vi "HFRR ADV v038 new software.vi"() -> ()   [LabVIEW 2025] (continued)
        n1697 = call <vilib>:"Clear Errors.vi"("error in (no error)"=w2110) -> ()  [unwired: 5 in, 2 out]
        n1698 = local write "Port 2a"(FALSE ("Port 2a")) -> ()
        n1699 = local read "Com Port 2"() -> (w2103:refnum<visa-resource-name>)
        "visa due" <- w2103
        n1700 = call-poly "VISA Configure Serial Port"("VISA resource name"=w2103, "timeout (10sec)"=w2114, "baud rate (9600)"=u32 250000 ("baud rate  2"), "data bits (8)"=u16 8 ("data bits  2"), "parity (0:none)"=w2113, "stop bits (10: 1 bit)"=w2115, "flow control (0:none)"=w2117) -> ("VISA resource name out"=w2118:refnum<visa-resource-name>, "error out"=w2119:errorcluster)  [unwired: 7 in]
        n1701 = flat-sequence {
          tunnel: w2118 -> [w2121]
          tunnel: w2119 -> [w2120]
          tunnel: [w2121] -> w2111
          tunnel: [w2120] -> w2104
          frame #0 {
            n1702 = Wait (ms)(milliseconds to wait=u32 50) -> ()  [unwired: 1 out]
          }
        }
        "Residual Due" <- ""
      }
    }
    "error out 9" <- w2045
    n1703 = local read "Quit"() -> (w2047:bool)
    "Error Due" <- w2052
  }
  n1704 = local write "FRICVALZ"(0.0 ("FRICVALZ")) -> ()
  n1705 = property on="RUN" class="Bool (strict)"("Visible"=TRUE) -> ()  [unwired: 2 in, 2 out]
  n1706 = while {
    tunnel: [w2136] -> _
    tunnel: [w2123] -> w54
    i -> [w2136]
    stop <- w2123 stop-if-true
    n1707 = local read "conststatus"() -> (w2127:dbl)
    n1708 = local read "Main Tab"() -> (w2125:T2)
    n1709 = local read "EDIT"() -> (w2142:bool)
    n1710 = local read "Rate"() -> (w2141:dbl)
    n1711 = case shown="True" w2142 {
      tunnel: [FALSE TRUE] -> _
      frame False {
      }
      frame True {
      }
    }
    n1712 = Equal?(x=w2125, y=T28."About" ("Main Tab")) -> (x = y?=w2134:bool)
    n1713 = Equal?(x=w2127, y=0.0) -> (x = y?=w2128:bool)
    n1714 = Divide(x=1.0, y=w2141) -> (x/y=w2137:dbl)
    "Time 2" <- w2137
    n1715 = case shown="True" w2128 {
      frame False {
      }
      frame True {
        # "C:\\WinDucom\\calibrate WO 2391.dcf"
        n1716 = local write "Lan flag"(22) -> ()
        n1717 = local write "conststatus"(10.0 ("rpm value : 2")) -> ()
        n1718 = String To Path(string="C:\\LAB-IQ\\calibrate WO 2465.dcf") -> (path=w2148:path)
        n1719 = Open/Create/Replace File "Open File"(file path (use dialog)=w2148) -> (refnum out=w2146:refnum<file>)  [unwired: 5 in, 2 out]
        n1720 = for {
          N: 23 -> [_]
          tunnel: w2146 -> [w2157]
          i -> [w2151]
          (unwired) TRUE ("line mode (F)")
          n1721 = Read from Text File "Read File"(file (use dialog)=w2157) -> (text=w2156:string)  [unwired: 3 in, 3 out]
          n1722 = Match Pattern(string=w2156, regular expression="]") -> (after substring=w2154:string)  [unwired: 1 in, 3 out]
          n1723 = String Subset(string=w2156, offset (0)=5, length (rest)=10 ("length (rest)")) -> (substring=w2149:string)
          n1724 = Fract/Exp String To Number(string=w2149) -> (number=w2150:dbl)  [unwired: 3 in, 1 out]
          n1725 = Match Pattern(string=w2154, regular expression="-") -> (before substring=w2152:string)  [unwired: 1 in, 3 out]
          n1726 = case shown="10" w2151 {
            tunnel: w2150 -> [_ _ _ _ _ _ _ _ _ _ w2164 _ _ _ _ _ _ _ _ _ _ _ _ _]
            tunnel: w2152 -> [_ _ _ _ w2160 w2161 w2162 _ _ _ _ _ _ _ _ _ _ _ _ _ w2165 w2166 w2167 _]
            frame 0 {
            }
            frame 1 {
            }
            frame 2 {
            }
            frame 3 {
            }
            frame 4 {
              n1727 = local write "Com Port 1"(w2160) -> ()
            }
            frame 5 {
              n1728 = local write "Com Port 2"(w2161) -> ()
              n1729 = local write "visa due"(w2161) -> ()
            }
            frame 6 {
              n1730 = String To Path(string=w2162) -> (path=w2163:path)
              n1731 = local write "File Path"(w2163) -> ()
              "String" <- w2162
            }
            frame 7 {
            }
            frame 8 {
            }
            frame 9 {
            }
            frame 10 {
              n1732 = local write "Language Selection"(w2164) -> ()
            }
            frame 11 {
            }
            frame 12 {
            }
            frame 13 {
            }
            frame 14 {
            }
            frame 15 {
            }
            frame 16 {
            }
            frame 17 {
            }
            frame 18 {
            }
            frame 21 {
            }
            frame 22 {
              n1733 = local write "Com Port 3"(w2165) -> ()
            }
            frame 20 {
              n1734 = local write "Camera Port :"(w2166) -> ()
            }
            frame 19 {
              n1735 = local write "C3 :"(w2167) -> ()
            }
            frame 23, Default {
            }
          }
        }
      }
    }
    n1736 = Select(t=u32 2500 ("milliseconds to wait"), s=w2134, f=u32 500 ("milliseconds to wait")) -> (s? t:f=w2132:u32)
    n1737 = Multiply(x=w2137, y=w2132) -> (x*y=w2139:dbl)
    n1738 = call "Elapsed Time2"("Time Target (s)"=w2139, "Auto Reset"=TRUE) -> ("Time has Elapsed"=w2129:bool)  [unwired: 10 in, 7 out]
    n1739 = case shown="True" w2129 {
      frame False {
      }
      frame True {
        n1740 = stacked-sequence {
          frame #0 {
            # "DATA PROCESSING"
            # "115 mV/N"
            n1741 = local read "Sample Temperature"() -> (w2170:dbl)
            n1742 = local read "RH Numeric:"() -> (→"Humidity ( %RH )" →"Hum":dbl)
            n1743 = local read "FRICVALZ"() -> (w2187:dbl)
            n1744 = local read "Friction"() -> (w2173:dbl)
            n1745 = call <vilib>:"Mean PtByPt.vi"("x"=w2170, "sample length"=100) -> ("mean"=w2169:dbl)  [unwired: 2 in, 1 out]
            "TEMP 2" <- w2169
            "TEMP 3" <- w2169
            n1746 = Subtract(x=w2173, y=w2187) -> (x-y=w2182:dbl)
            "FF 2" <- w2182
            "FF 4" <- w2182
            n1747 = local read "Ambient Temperature"() -> (→"AIR TEMP":dbl)
            n1748 = local read "TEMP"() -> (w2186:dbl)
            n1749 = local write "FF 3"(w2182) -> ()
            n1750 = Compound Arithmetic op=OR("FRICVALZ 4", "FRICVALZ 3", "FRICVALZ 2") -> (w2178:bool)
            n1751 = case shown="True" w2178 {
              tunnel: w2173 -> [_ w2193]
              frame False {
              }
              frame True {
                w2192 = FALSE ("FRICVALZ")
                n1752 = local write "FRICVALZ 3"(w2192) -> ()
                n1753 = local write "FRICVALZ 2"(w2192) -> ()
                n1754 = local write "FRICVALZ 4"(w2192) -> ()
                "FRICVALZ" <- w2193
              }
            }
            n1755 = Not A Number/Path/Refnum?(number/path/refnum=w2186) -> (NaN/Path/Refnum?=w2185:bool)
            n1756 = Not A Number/Path/Refnum?(number/path/refnum=w2182) -> (NaN/Path/Refnum?=w2184:bool)
            n1757 = Divide(x=w2182, y=1.96) -> (x/y=w2179:dbl)
            n1758 = Compound Arithmetic op=OR(w2185, w2184) -> (w2183:bool)
            n1759 = Not A Number/Path/Refnum?(number/path/refnum=w2179) -> (NaN/Path/Refnum?=w2180:bool)
            n1760 = case shown="True" w2183 {
              frame False {
              }
              frame True {
                n1761 = local write "TEMP"(0.0 ("TEMP")) -> ()
                n1762 = local write "FF 2"(0.0 ("FF 2")) -> ()
                n1763 = local write "reinit"(TRUE ("reinit")) -> ()
              }
            }
            n1764 = local write "TEMP"(w2169) -> ()
            n1765 = Select(t=0.0, s=w2180, f=w2179) -> (s? t:f=w2172:dbl)
            "COF 2" <- w2172
            n1766 = local write "COF 3"(w2172) -> ()
          }
        }
      }
    }
    n1767 = Wait (ms)(milliseconds to wait=u32 50) -> ()  [unwired: 1 out]
    n1768 = local read "Quit"() -> (w2123:bool)
    "Rate" <- 2500.0 ("No of Samples")
  }
  n1769 = while {
    tunnel: [w2213] -> _
    tunnel: [w2196] -> w56
    tunnel: w1 -> [_]
    i -> [w2213]
    stop <- w2196 stop-if-true
    # "C:\\LAB-IQ-NXT\\Scar View.exe"
    n1770 = local read "OK Button 16"() -> (w2203:bool)
    n1771 = local read "Main Tab"() -> (w2197:T2)
    n1772 = local read "service 3"() -> (w2198:bool)
    n1773 = local read "OPEN 6"() -> (w2200:bool)
    n1774 = local read "EDIT 2"() -> (w2202:bool)
    n1775 = flat-sequence {
      frame #0 {
        n1776 = stacked-sequence {
          frame #0 {
            n1777 = local read "EDIT"() -> (w2691:bool)
            n1778 = case shown="False" w2691 {
              tunnel: [u8 2 ("Disabled") u8 0 ("Disabled")] -> _
              frame False {
                w2693 = FALSE
                n1779 = local write "Password"("") -> ()
                n1780 = local write "x = y?"(w2693) -> ()
                n1781 = property on="Password" class="Str"("Visible"=w2693) -> ()  [unwired: 2 in, 2 out]
              }
              frame True {
                n1782 = property on="Password" class="Str"("Visible"=TRUE) -> ()  [unwired: 2 in, 2 out]
              }
            }
            "dipl pwd" <- "@143$\n" ("dipl pwd")
          }
          frame #1 {
          }
          frame #2 {
          }
          frame #3 {
          }
          frame #4 {
            n1783 = String To Byte Array(string="Password") -> (unsigned byte array=w2704:u8[])
            n1784 = Search 1D Array(1D array=w2704, element=u8 10) -> (index of element=w2702:i32)  [unwired: 1 in]
            n1785 = Index Array(array=w2704, index=w2702) -> (element=w2703:u8)
            n1786 = Equal?(x=w2703, y=10) -> (x = y?=w2699:bool)
            n1787 = case shown="True" w2699 {
              frame False {
              }
              frame True {
                # "password"
                # "password"
                n1788 = local read "Password"() -> (w2716:string)
                n1789 = String To Byte Array(string=w2716) -> (unsigned byte array=w2719:u8[])
                n1790 = String To Byte Array(string="@143$\n") -> (unsigned byte array=w2706:u8[])
                n1791 = Array Size(array=w2719) -> (size(s)=w2715:i32)
                n1792 = Array Size(array=w2706) -> (size(s)=w2711:i32)
                n1793 = for {
                  N: w2715 -> [_]
                  tunnel: w2719 -> [w2732]
                  tunnel: [w2730] -> w2720 mode=indexing
                  tunnel: w2715 -> [w2727]
                  i -> [w2728]
                  n1794 = Decrement(x=w2727) -> (x-1=w2726:i32)
                  n1795 = Index Array(array=w2732, index=w2728) -> (element=w2731:u8)
                  n1796 = Equal?(x=w2728, y=w2726) -> (x = y?=w2725:bool)
                  n1797 = Number To Decimal String(number=w2731) -> (decimal integer string=w2729:string)  [unwired: 1 in]
                  n1798 = Select(t="", s=w2725, f="\r") -> (s? t:f=w2722:string)
                  n1799 = Concatenate Strings(w2729, w2722) -> (w2730:string)
                }
                n1800 = for {
                  N: w2711 -> [_]
                  tunnel: w2706 -> [w2743]
                  tunnel: [w2741] -> w2709 mode=indexing
                  tunnel: w2711 -> [w2738]
                  i -> [w2739]
                  n1801 = Decrement(x=w2738) -> (x-1=w2737:i32)
                  n1802 = Index Array(array=w2743, index=w2739) -> (element=w2742:u8)
                  n1803 = Equal?(x=w2739, y=w2737) -> (x = y?=w2736:bool)
                  n1804 = Number To Decimal String(number=w2742) -> (decimal integer string=w2740:string)  [unwired: 1 in]
                  n1805 = Select(t="", s=w2736, f="\r") -> (s? t:f=w2733:string)
                  n1806 = Concatenate Strings(w2740, w2733) -> (w2741:string)
                }
                n1807 = local read "file path"() -> (w2705:path)
                n1808 = call <vilib>:"Read Characters From File.vi"("file path (dialog if empty)"=w2705) -> ("character string"=w2718:string)  [unwired: 5 in, 3 out]
                "string" <- w2718
                n1809 = flat-sequence {
                  tunnel: [w2721] -> _
                  frame #0 {
                    w2721 = ""
                    n1810 = local write "Password"(w2721) -> ()
                  }
                }
                n1811 = Concatenate Strings(w2709) -> (w2710:string)
                n1812 = Concatenate Strings(w2718) -> (w2717:string)
                n1813 = Concatenate Strings(w2720) -> (w2713:string)
                n1814 = Equal?(x=w2713, y=w2717) -> (x = y?=w2708:bool)
                n1815 = Equal?(x=w2713, y=w2710) -> (x = y?=w2714:bool)
                n1816 = Or(x=w2708, y=w2714) -> (x .or. y?=→"x = y?":bool)
              }
            }
          }
        }
        n1817 = local read "x = y?"() -> (w2689:bool)
        n1818 = And(x="EDIT", y=w2689) -> (x .and. y?=w2687:bool)
        n1819 = case shown="True" w2687 {
          tunnel: [u8 2 ("Disabled") u8 0 ("Disabled")] -> w2686
          tunnel: [w2893 TRUE ("Visible")] -> w2685
          frame False {
            w2893 = FALSE ("Visible")
            n1820 = local write "EDIT 2"(w2893) -> ()
          }
          frame True {
          }
        }
        n1821 = case shown="True" "SAVE" {
          frame False {
          }
          frame True {
            n1822 = stacked-sequence {
              seq-local: [w2748 _ _] -> [_ w2889 _]
              frame #0 {
                w2744 = 0.0 ("number")
                w2745 = 0.0 ("number")
                (unwired) i16 5 ("precision (6)")
                # "[CH1]    - FF\n[CH2]   - TEMPERATURE\n[CH3]    - Humidity\n[CH4]    - AIR TEMP\n[CH5]\\- Visa Uno\n[CH6] \\- Visa Due\n[CH7]  \\- file path\n[CH8]   - Displacement Gain\n[CHA]   - Stroke Gain\n[CHB]   - Stroke PID Gain\n[CHC]   -Language Selection\n[CHD]   -Power +\n[CHE]   -Power_\n[CHF]   -Heater\n[CHG]   -Humidity Wet\n[CHH]   -Humidity Dry\n[CHI]   -Integral Time"
                n1823 = local read "Language Selection"() -> (w2791:enum16{"English", "Russian"})
                n1824 = Path To String(path="File Path") -> (string=w2807:string)
                n1825 = Number To Fractional String(number=w2744, width (-)=i16 10 ("precision (6)"), precision (6)=i16 5) -> (F-format string=w2798:string)  [unwired: 1 in]
                n1826 = Number To Fractional String(number=w2791, width (-)=i16 10 ("precision (6)"), precision (6)=i16 5) -> (F-format string=w2787:string)  [unwired: 1 in]
                n1827 = Number To Fractional String(number=w2745, width (-)=i16 10 ("precision (6)"), precision (6)=i16 5) -> (F-format string=w2781:string)  [unwired: 1 in]
                n1828 = Number To Fractional String(number=w2745, width (-)=i16 10 ("precision (6)"), precision (6)=i16 5) -> (F-format string=w2778:string)  [unwired: 1 in]
                n1829 = Number To Fractional String(number=w2745, width (-)=i16 10 ("precision (6)"), precision (6)=i16 5) -> (F-format string=w2773:string)  [unwired: 1 in]
                n1830 = Number To Fractional String(number=w2745, width (-)=i16 10 ("precision (6)"), precision (6)=i16 5) -> (F-format string=w2770:string)  [unwired: 1 in]
                n1831 = Number To Fractional String(number=w2745, width (-)=i16 10 ("precision (6)"), precision (6)=i16 5) -> (F-format string=w2765:string)  [unwired: 1 in]
                n1832 = local read "Com Port 1"() -> (w2747:refnum<visa-resource-name>)
                n1833 = local read "Com Port 2"() -> (w2746:refnum<visa-resource-name>)
                n1834 = Concatenate Strings(w2807, "\\" ("string")) -> (w2806:string)
                n1835 = Number To Fractional String(number=w2744, width (-)=i16 10 ("precision (6)"), precision (6)=i16 5) -> (F-format string=w2839:string)  [unwired: 1 in]
                n1836 = Number To Fractional String(number=w2744, width (-)=i16 10 ("precision (6)"), precision (6)=i16 5) -> (F-format string=w2838:string)  [unwired: 1 in]
                n1837 = Number To Fractional String(number=w2744, width (-)=i16 10 ("precision (6)"), precision (6)=i16 5) -> (F-format string=w2832:string)  [unwired: 1 in]
                n1838 = Number To Fractional String(number=w2744, width (-)=i16 10 ("precision (6)"), precision (6)=i16 5) -> (F-format string=w2826:string)  [unwired: 1 in]
                n1839 = Number To Fractional String(number=w2744, width (-)=i16 10 ("precision (6)"), precision (6)=i16 5) -> (F-format string=w2799:string)  [unwired: 1 in]
                n1840 = Concatenate Strings("[CHA]" ("string"), w2798, "- Stroke Gain" ("string"), "\r") -> (w2792:string)
                n1841 = Concatenate Strings("[CHC]" ("string"), w2787, "-Language Selection" ("string"), "\r") -> (w2784:string)
                n1842 = Concatenate Strings("[CHD]" ("string"), w2781, "-Power +" ("string"), "\r") -> (w2763:string)
                n1843 = Concatenate Strings("[CHG]" ("string"), w2770, "-Humidity Wet" ("string"), "\r") -> (w2760:string)
                n1844 = Concatenate Strings("[CHH]" ("string"), w2765, "-Humidity Dry" ("string"), "\r") -> (w2759:string)
                n1845 = Concatenate Strings("[CH1]" ("string"), w2839, " - FF" ("string"), "\r") -> (w2837:string)
                n1846 = Concatenate Strings("[CH2]" ("string"), w2838, " - TEMPERATURE" ("string"), "\r") -> (w2836:string)
                n1847 = Concatenate Strings("[CH3]" ("string"), w2832, " - Humidity" ("string"), "\r") -> (w2829:string)
                n1848 = Concatenate Strings("[CH4]" ("string"), w2826, " - AIR TEMP" ("string"), "\r") -> (w2822:string)
                n1849 = Concatenate Strings("[CH5]" ("string"), w2747, "- Visa Uno" ("string"), "\r") -> (w2815:string)
                n1850 = Concatenate Strings("[CH6]" ("string"), w2746, "- Visa Due" ("string"), "\r") -> (w2810:string)
                n1851 = Concatenate Strings("[CH7]" ("string"), w2806, "- file path" ("string"), "\r") -> (w2809:string)
                n1852 = Concatenate Strings("[CH8]" ("string"), w2799, "- Displacement Gain" ("string"), "\r") -> (w2802:string)
                n1853 = Concatenate Strings("[CHE]" ("string"), w2778, "-Power_" ("string"), "\r") -> (w2762:string)
                n1854 = Concatenate Strings("[CHF]" ("string"), w2773, "-Heater" ("string"), "\r") -> (w2761:string)
                n1855 = Concatenate Strings(w2837, w2836, w2829, w2822, w2815, w2810, w2809, w2802, w2792, w2784, w2763, w2762, w2761, w2760, w2759) -> (w2748:string)
                "gain" <- w2748
              }
              frame #1 {
                w2850 = 0.0 ("number")
                n1856 = local read "Camera Port :"() -> (w2853:string)
                n1857 = local read "C3 :"() -> (w2861:refnum<visa-resource-name>)
                n1858 = local read "Com Port 3"() -> (w2862:refnum<visa-resource-name>)
                n1859 = Concatenate Strings("[CH8]" ("string"), w2853, "- Visa Camera" ("string"), "\r") -> (w2852:string)
                n1860 = Concatenate Strings("[CH7]" ("string"), w2861, "- Visa Humidity" ("string"), "\r") -> (w2857:string)
                n1861 = Number To Fractional String(number=w2850, width (-)=i16 10 ("precision (6)"), precision (6)=i16 5) -> (F-format string=w2877:string)  [unwired: 1 in]
                n1862 = Concatenate Strings("[CHL]" ("string"), w2862, "- Visa humid" ("string"), "\r") -> (w2865:string)
                n1863 = Number To Fractional String(number=w2850, width (-)=i16 10 ("precision (6)"), precision (6)=i16 5) -> (F-format string=w2884:string)  [unwired: 1 in]
                n1864 = Concatenate Strings("[CHK]" ("string"), w2877, "-TEMP INTERCEPT" ("string"), "\r") -> (w2873:string)
                n1865 = Concatenate Strings("[SNO]" ("string"), "" ("string"), "-" ("string"), "\r") -> (w2870:string)
                n1866 = Concatenate Strings("[CHJ]" ("string"), w2884, "-AIR TEMP INTERCEPT" ("string"), "\r") -> (w2874:string)
                n1867 = String To Path(string="C:\\LAB-IQ\\calibrate WO 2465.dcf") -> (path=w2863:path)
                n1868 = Concatenate Strings(w2889, w2874, w2873, w2870, w2865, w2857, w2852) -> (w2888:string)
                n1869 = call <vilib>:"Write Characters To File.vi"("append to file? (new file:F)"=FALSE, "character string"=w2888, "file path (dialog if empty)"=w2863) -> ()  [unwired: 2 in, 1 out]
              }
              frame #2 {
                n1870 = local write "Lan flag"(0.0 ("Lan flag")) -> ()
                n1871 = local write "conststatus"(0.0 ("rpm value : 2")) -> ()
                n1872 = local write "SAVE"(FALSE ("OK Button 14")) -> ()
              }
            }
          }
        }
        n1873 = property on="EDIT 2" class="Bool (strict)"("Visible"=w2685) -> ()  [unwired: 2 in, 2 out]
        n1874 = property on="SAVE" class="Bool (strict)"("Visible"=w2685) -> ()  [unwired: 2 in, 2 out]
        n1875 = property on="visa due" class="CmbBox"("Disabled"=w2686) -> ()  [unwired: 2 in, 2 out]
        n1876 = property on="File Path" class="Path"("Disabled"=w2686) -> ()  [unwired: 2 in, 2 out]
        n1877 = property on="Language Selection" class="Enum (strict)"("Visible"=w2685) -> ()  [unwired: 2 in, 2 out]
        n1878 = property on="SPEED OUT:" class="DigNum (strict)"("Disabled"=w2686) -> ()  [unwired: 2 in, 2 out]
      }
    }
    n1879 = local read "RUN"() -> (w2212:bool)
    n1880 = local read "RUN"() -> (w2210:bool)
    n1881 = case shown="True" "EDIT 3" {
      frame False {
      }
      frame True {
        n1882 = local write "EDIT 3"(FALSE ("EDIT 3")) -> ()
        n1883 = local write "Main Tab"(T2."About" ("Main Tab")) -> ()
      }
    }
    n1884 = case shown="False" w2212 {
      frame False {
        n1885 = local read "stopT"() -> (w2900:bool)
        n1886 = case shown="True" w2900 {
          frame False {
          }
          frame True {
            n1887 = local write "stopT"(FALSE) -> ()
          }
        }
      }
      frame True {
        "stopT" <- TRUE
      }
    }
    n1888 = case shown="False" w2210 {
      frame False {
      }
      frame True {
      }
    }
    n1889 = case shown="True" w2202 {
      frame False {
        n1890 = property on="Password 2" class="Str"("Visible"=FALSE) -> ()  [unwired: 2 in, 2 out]
        n1891 = local write "Password 2"("" ("Password")) -> ()
      }
      frame True {
        n1892 = property on="Password 2" class="Str"("Visible"=TRUE) -> ()  [unwired: 2 in, 2 out]
        n1893 = Equal?(x="Password 2", y="HFRR1234") -> (x = y?=w2225:bool)
        n1894 = case shown="True" w2225 {
          tunnel: "Password 2" -> [w2228 _]
          frame False {
            n1895 = String Length(string=w2228) -> (length=w2229:i32)
            n1896 = Greater Than 0?(x=w2229) -> (x > 0?=w2227:bool)
            n1897 = case shown="False" w2227 {
              frame False {
                n1898 = property on="Password 2" class="Str"("Caption.Text"="Password (Advance Setting)") -> ()  [unwired: 2 in, 2 out]
              }
              frame True {
                n1899 = property on="Password 2" class="Str"("Caption.Text"="Incorrect Password!") -> ()  [unwired: 2 in, 2 out]
              }
            }
          }
          frame True {
            n1900 = local write "EDIT 2"(FALSE ("EDIT 2")) -> ()
            n1901 = local write "Password 2"("" ("Password")) -> ()
            n1902 = local write "Main Tab"(T2."Advance" ("Main Tab")) -> ()
            n1903 = local write "Main Dashboard Buttons"(T1."Advance" ("Main Dashboard Buttons")) -> ()
          }
        }
      }
    }
    n1904 = case shown="True" "Prog Uno" {
      frame False {
      }
      frame True {
        n1905 = stacked-sequence {
          frame #0 {
            n1906 = Delete(path (use dialog)=path "C:/LAB-IQ-NXT/UNOCOMPILE.bat" ("working directory")) -> ()  [unwired: 4 in, 3 out]
          }
          frame #1 {
            n1907 = local read "Com Port 1"() -> (w2667:refnum<visa-resource-name>)
            n1908 = Concatenate Strings("cmd.exe /c \"mode " ("command line"), w2667, ":1200,n,8,1\"\n" ("command line")) -> (w2672:string)
            n1909 = Concatenate Strings(w2672, "CD\\\nCD WinDucom\navrdude -C avrdude.conf -v -patmega328p -carduino -P" ("command line"), w2667, " -b115200 -D -Uflash:w:UNO_V20.hex:i\n" ("command line"), "\r") -> (w2674:string)
            "STR" <- w2674
            n1910 = call <vilib>:"Write Characters To File.vi"("append to file? (new file:F)"=FALSE, "character string"=w2674, "file path (dialog if empty)"=path "C:/LAB-IQ/UNOCOMPILE.bat" ("working directory")) -> ()  [unwired: 2 in, 1 out]
          }
          frame #2 {
            n1911 = disable-structure shown="Disabled" {
              frame Disabled {
                w2678 = "cmd.exe  /c \"C:\\LAB-IQ-NXT\\UNOCOMPILE.bat\"" ("string")
                n1912 = local write "Prog Uno"(FALSE ("run minimized? (F)")) -> ()
                n1913 = call <vilib>:"System Exec.vi"("expected output size  (4096)"=u32 65535, "run minimized? (F)"=FALSE, "wait until completion? (T)"=TRUE ("run minimized? (F)"), "working directory"=path "C:/LAB-IQ-NXT", "standard input"=w2678, "command line"=w2678) -> ("error out"=w2677:errorcluster, "standard output"=→"String 42":string)  [unwired: 2 in, 2 out]
                "error out 3" <- w2677
                n1914 = flat-sequence {
                  tunnel: w2677 -> [_]
                  frame #0 {
                  }
                }
              }
              frame Enabled {
              }
            }
          }
        }
      }
    }
    n1915 = case shown="\"ISO 12156\"" "TEST STANDARD" {
      frame "ASTM D6079", Default {
        w2647 = 50.0 ("Hz")
        w2648 = 53.0 ("Set Rh")
        w2650 = 1.0 ("Set Strk")
        w2649 = 60.0 ("Set Temp")
        # "astm hide"
        n1916 = local write "NORMAL LOAD"(200.0 ("NORMAL LOAD")) -> ()
        n1917 = local write "Set Strk"(w2650) -> ()
        n1918 = local write "Set Hz"(w2647) -> ()
        n1919 = local write "Set Temp"(w2649) -> ()
        n1920 = local write "Set Rh"(w2648) -> ()
        n1921 = local write "test time"(75.0 ("test time")) -> ()
        n1922 = local write "Set Stroke:"(w2650) -> ()
        n1923 = local write "Set Humidity:"(w2648) -> ()
        n1924 = local write "Set Frequency:"(w2647) -> ()
        n1925 = local write "Set Temperature:"(w2649) -> ()
        "Test Standard" <- "ASTM D6079" ("Test Standard 2")
      }
      frame "ISO 12156" {
        n1926 = local write "Set Strk"(1.0 ("Set Strk")) -> ()
        n1927 = local write "NORMAL LOAD"(200.0 ("NORMAL LOAD")) -> ()
        n1928 = local write "Set Temp"(60.0 ("Set Temp")) -> ()
        n1929 = local write "test time"(75.0 ("test time")) -> ()
        n1930 = local write "Set Hz"(50.0 ("Hz")) -> ()
        n1931 = local write "Set Rh"(53.0 ("Set Rh")) -> ()
      }
      frame "CEC F-096-A-06" {
        n1932 = local write "Set Strk"(1.0 ("Set Strk")) -> ()
        n1933 = local write "NORMAL LOAD"(200.0 ("NORMAL LOAD")) -> ()
        n1934 = local write "Set Temp"(60.0 ("Set Temp")) -> ()
        n1935 = local write "test time"(75.0 ("test time")) -> ()
        n1936 = local write "Set Hz"(50.0 ("Hz")) -> ()
        n1937 = local write "Set Rh"(53.0 ("Set Rh")) -> ()
      }
      frame "Custom" {
      }
    }
    n1938 = Or(x=w2200, y=w2198) -> (x .or. y?=w2199:bool)
    n1939 = case shown="\"About\"" w2197 {
      tunnel: [T28."Acquire" ("Main Tab") T28."Compare Files" ("Main Tab") T28."About" ("Main Tab")] -> w2208
      frame "Acquire", Default {
      }
      frame "Compare Files" {
      }
      frame "About" {
      }
    }
    n1940 = Or(x=w2203, y="OPEN") -> (x .or. y?=w2204:bool)
    n1941 = case shown="True" w2204 {
      tunnel: w2203 -> [_ w2236]
      frame False {
      }
      frame True {
        n1942 = stacked-sequence {
          tunnel: w2236 -> [_ w2303 _ _]
          frame #0 {
            w2252 = "  " ("String 6")
            n1943 = local write "OPEN"(FALSE ("open")) -> ()
            n1944 = local read "string1 2"() -> (w2240:string)
            n1945 = local read "string1 3"() -> (w2239:string)
            n1946 = local read "string1 4"() -> (w2238:string)
            n1947 = property on="OPEN" class="Bool (strict)"("Visible"=FALSE) -> ()  [unwired: 2 in, 2 out]
            n1948 = local write "String 6"(w2252) -> ()
            n1949 = local write "String 7"(w2252) -> ()
            n1950 = local write "String 8"(w2252) -> ()
            n1951 = local write "String 12"(w2252) -> ()
            n1952 = local read "OK Button 16"() -> (w2237:bool)
            n1953 = String To Path(string=w2240) -> (path=w2248:path)
            n1954 = String To Path(string=w2239) -> (path=w2247:path)
            n1955 = String To Path(string=w2238) -> (path=w2246:path)
            n1956 = case shown="True" w2237 {
              tunnel: [w2253 w2254] -> w2241
              frame False {
                n1957 = local read "string1"() -> (w2253:string)
              }
              frame True {
                n1958 = local read "String Indicator 4"() -> (w2254:string)
              }
            }
            n1959 = Open/Create/Replace File "Open File"(file path (use dialog)=w2248) -> (refnum out=w2244:refnum<file>)  [unwired: 5 in, 2 out]
            n1960 = Open/Create/Replace File "Open File"(file path (use dialog)=w2247) -> (refnum out=w2243:refnum<file>)  [unwired: 5 in, 2 out]
            n1961 = Open/Create/Replace File "Open File"(file path (use dialog)=w2246) -> (refnum out=w2242:refnum<file>)  [unwired: 5 in, 2 out]
            n1962 = while {
              tunnel: w2244 -> [w2266]
              i -> [w2262]
              stop <- w2261 continue-if-true
              (unwired) TRUE ("line mode (F)")
              n1963 = Read from Text File "Read File"(file (use dialog)=w2266) -> (text=w2263:string)  [unwired: 3 in, 3 out]
              n1964 = local write "Numeric 11"(w2262) -> ()
              n1965 = String Length(string=w2263) -> (length=w2265:i32)
              n1966 = Greater?(x=w2265, y=1) -> (0:w2261:bool)
            }
            n1967 = while {
              tunnel: w2243 -> [w2272]
              i -> [w2268]
              stop <- w2267 continue-if-true
              (unwired) TRUE ("line mode (F)")
              n1968 = Read from Text File "Read File"(file (use dialog)=w2272) -> (text=w2269:string)  [unwired: 3 in, 3 out]
              n1969 = local write "Numeric 12"(w2268) -> ()
              n1970 = String Length(string=w2269) -> (length=w2271:i32)
              n1971 = Greater?(x=w2271, y=1) -> (0:w2267:bool)
            }
            n1972 = while {
              tunnel: w2242 -> [w2278]
              i -> [w2274]
              stop <- w2273 continue-if-true
              (unwired) TRUE ("line mode (F)")
              n1973 = Read from Text File "Read File"(file (use dialog)=w2278) -> (text=w2275:string)  [unwired: 3 in, 3 out]
              n1974 = local write "Numeric 13"(w2274) -> ()
              n1975 = String Length(string=w2275) -> (length=w2277:i32)
              n1976 = Greater?(x=w2277, y=1) -> (0:w2273:bool)
            }
            n1977 = String To Path(string=w2241) -> (path=w2249:path)
            n1978 = Open/Create/Replace File "Open File"(file path (use dialog)=w2249) -> (refnum out=w2245:refnum<file>)  [unwired: 5 in, 2 out]
            n1979 = while {
              tunnel: w2245 -> [w2260]
              i -> [w2256]
              stop <- w2255 continue-if-true
              (unwired) TRUE ("line mode (F)")
              n1980 = Read from Text File "Read File"(file (use dialog)=w2260) -> (text=w2257:string)  [unwired: 3 in, 3 out]
              n1981 = local write "Numeric 8"(w2256) -> ()
              n1982 = String Length(string=w2257) -> (length=w2259:i32)
              n1983 = Greater?(x=w2259, y=1) -> (0:w2255:bool)
            }
          }
          frame #1 {
            w2430 = FALSE ("ACTUAL   MERGE")
            # "Sample Temp"
            # "ECR"
            # "COF"
            # "Time\nCOF\nFF\nTemp"
            n1984 = case shown="True" w2303 {
              tunnel: [w2450 w2451] -> w2304
              frame False {
                n1985 = local read "string1"() -> (w2450:string)
              }
              frame True {
                n1986 = local read "String Indicator 4"() -> (w2451:string)
              }
            }
            n1987 = local read "string1 3"() -> (w2348:string)
            n1988 = String To Path(string=w2304) -> (path=w2435:path)
            n1989 = String To Path(string=w2348) -> (path=w2446:path)
            n1990 = local read "Numeric 12"() -> (w2432:i32)
            n1991 = local read "Numeric 8"() -> (w2434:i32)
            n1992 = local read "string1 2"() -> (w2349:string)
            n1993 = local read "string1 4"() -> (w2347:string)
            n1994 = Open/Create/Replace File "Open File"(file path (use dialog)=w2435) -> (refnum out=w2449:refnum<file>, error out=w2448:errorcluster)  [unwired: 5 in, 1 out]
            n1995 = Open/Create/Replace File "Open File"(file path (use dialog)=w2446) -> (refnum out=w2442:refnum<file>, error out=w2443:errorcluster)  [unwired: 5 in, 1 out]
            n1996 = for {
              N: w2434 -> [_]
              tunnel: w2449 -> [w2597]
              tunnel: w2448 -> [w2596]
              tunnel: [w2586] -> w2361 mode=indexing
              tunnel: [w2584] -> w2418 mode=indexing
              tunnel: [w2585] -> w2413 mode=indexing
              tunnel: w2430 -> [_]
              tunnel: [w2578] -> w2415 mode=indexing
              tunnel: [w2574] -> w2384 mode=indexing
              tunnel: [w2570] -> w2359 mode=indexing
              tunnel: [w2566] -> w2340 mode=indexing
              tunnel: [w2561] -> w2300 mode=indexing
              (unwired) TRUE ("line mode (F)")
              # "freq"
              # "Stroke"
              # "Time"
              # "CoF"
              # "Humidity"
              # "Temp"
              # "Air Temp"
              # "ECR"
              n1997 = Read from Text File "Read File"(file (use dialog)=w2597, error in=w2596) -> (text=w2562:string)  [unwired: 2 in, 3 out]
              n1998 = local write "String 6"(w2562) -> ()
              n1999 = String Subset(string=w2562, offset (0)=0, length (rest)=14 ("length (rest)")) -> (substring=w2590:string)
              n2000 = String Subset(string=w2562, offset (0)=35, length (rest)=9 ("length (rest)")) -> (substring=w2587:string)
              n2001 = String Subset(string=w2562, offset (0)=15, length (rest)=9 ("length (rest)")) -> (substring=w2593:string)
              n2002 = Fract/Exp String To Number(string=w2590) -> (number=w2586:dbl)  [unwired: 3 in, 1 out]
              n2003 = Fract/Exp String To Number(string=w2587) -> (number=w2585:dbl)  [unwired: 3 in, 1 out]
              n2004 = Fract/Exp String To Number(string=w2593) -> (number=w2584:dbl)  [unwired: 3 in, 1 out]
              n2005 = String Subset(string=w2562, offset (0)=85, length (rest)=9 ("length (rest)")) -> (substring=w2563:string)
              n2006 = String Subset(string=w2562, offset (0)=25, length (rest)=9 ("length (rest)")) -> (substring=w2569:string)
              n2007 = String Subset(string=w2562, offset (0)=55, length (rest)=9 ("length (rest)")) -> (substring=w2571:string)
              n2008 = String Subset(string=w2562, offset (0)=45, length (rest)=9 ("length (rest)")) -> (substring=w2577:string)
              n2009 = String Subset(string=w2562, offset (0)=65, length (rest)=9 ("length (rest)")) -> (substring=w2583:string)
              n2010 = Fract/Exp String To Number(string=w2569) -> (number=w2566:dbl)  [unwired: 3 in, 1 out]
              n2011 = Fract/Exp String To Number(string=w2563) -> (number=w2561:dbl)  [unwired: 3 in, 1 out]
              n2012 = Fract/Exp String To Number(string=w2571) -> (number=w2570:dbl)  [unwired: 3 in, 1 out]
              n2013 = Fract/Exp String To Number(string=w2577) -> (number=w2574:dbl)  [unwired: 3 in, 1 out]
              n2014 = Fract/Exp String To Number(string=w2583) -> (number=w2580:dbl)  [unwired: 3 in, 1 out]
              n2015 = Add(x=w2580, y=0.0) -> (x+y=w2578:dbl)
            }
            n2016 = for {
              N: w2432 -> [_]
              tunnel: w2443 -> [w2523]
              tunnel: w2442 -> [w2522]
              tunnel: [w2512] -> w2401 mode=indexing
              tunnel: [w2510] -> w2399 mode=indexing
              tunnel: [w2511] -> w2395 mode=indexing
              tunnel: w2430 -> [_]
              tunnel: [w2504] -> w2397 mode=indexing
              tunnel: [w2500] -> w2379 mode=indexing
              tunnel: [w2496] -> w2355 mode=indexing
              tunnel: [w2493] -> w2336 mode=indexing
              tunnel: [w2489] -> w2295 mode=indexing
              (unwired) 9 ("length (rest)")
              (unwired) 9 ("length (rest)")
              (unwired) TRUE ("line mode (F)")
              n2017 = Read from Text File "Read File"(file (use dialog)=w2522, error in=w2523) -> (text=w2490:string)  [unwired: 2 in, 3 out]
              n2018 = local write "String 8"(w2490) -> ()
              n2019 = String Subset(string=w2490, offset (0)=85) -> (substring=w2492:string)  [unwired: 1 in]
              n2020 = String Subset(string=w2490, offset (0)=35, length (rest)=9 ("length (rest)")) -> (substring=w2513:string)
              n2021 = String Subset(string=w2490, offset (0)=55, length (rest)=9 ("length (rest)")) -> (substring=w2498:string)
              n2022 = String Subset(string=w2490, offset (0)=25) -> (substring=w2494:string)  [unwired: 1 in]
              n2023 = String Subset(string=w2490, offset (0)=15, length (rest)=9 ("length (rest)")) -> (substring=w2519:string)
              n2024 = String Subset(string=w2490, offset (0)=0, length (rest)=14 ("length (rest)")) -> (substring=w2516:string)
              n2025 = String Subset(string=w2490, offset (0)=45, length (rest)=9 ("length (rest)")) -> (substring=w2503:string)
              n2026 = String Subset(string=w2490, offset (0)=65, length (rest)=9 ("length (rest)")) -> (substring=w2509:string)
              n2027 = Fract/Exp String To Number(string=w2492) -> (number=w2489:dbl)  [unwired: 3 in, 1 out]
              n2028 = Fract/Exp String To Number(string=w2513) -> (number=w2511:dbl)  [unwired: 3 in, 1 out]
              n2029 = Fract/Exp String To Number(string=w2498) -> (number=w2496:dbl)  [unwired: 3 in, 1 out]
              n2030 = Fract/Exp String To Number(string=w2494) -> (number=w2493:dbl)  [unwired: 3 in, 1 out]
              n2031 = Fract/Exp String To Number(string=w2519) -> (number=w2510:dbl)  [unwired: 3 in, 1 out]
              n2032 = Fract/Exp String To Number(string=w2516) -> (number=w2512:dbl)  [unwired: 3 in, 1 out]
              n2033 = Fract/Exp String To Number(string=w2503) -> (number=w2500:dbl)  [unwired: 3 in, 1 out]
              n2034 = Fract/Exp String To Number(string=w2509) -> (number=w2506:dbl)  [unwired: 3 in, 1 out]
              n2035 = Add(x=w2506, y=0.0) -> (x+y=w2504:dbl)
            }
            n2036 = String To Path(string=w2349) -> (path=w2447:path)
            n2037 = String To Path(string=w2347) -> (path=w2441:path)
            n2038 = local read "Numeric 11"() -> (w2431:i32)
            n2039 = local read "Numeric 13"() -> (w2433:i32)
            n2040 = Open/Create/Replace File "Open File"(file path (use dialog)=w2447) -> (refnum out=w2445:refnum<file>, error out=w2444:errorcluster)  [unwired: 5 in, 1 out]
            n2041 = Open/Create/Replace File "Open File"(file path (use dialog)=w2441) -> (refnum out=w2440:refnum<file>, error out=w2439:errorcluster)  [unwired: 5 in, 1 out]
            n2042 = for {
              N: w2431 -> [_]
              tunnel: w2445 -> [w2560]
              tunnel: w2444 -> [w2559]
              tunnel: [w2549] -> w2411 mode=indexing
              tunnel: [w2547] -> w2409 mode=indexing
              tunnel: [w2548] -> w2404 mode=indexing
              tunnel: w2430 -> [_]
              tunnel: [w2541] -> w2406 mode=indexing
              tunnel: [w2537] -> w2382 mode=indexing
              tunnel: [w2533] -> w2357 mode=indexing
              tunnel: [w2529] -> w2338 mode=indexing
              tunnel: [w2524] -> w2296 mode=indexing
              (unwired) TRUE ("line mode (F)")
              n2043 = Read from Text File "Read File"(file (use dialog)=w2560, error in=w2559) -> (text=w2525:string)  [unwired: 2 in, 3 out]
              n2044 = local write "String 7"(w2525) -> ()
              n2045 = String Subset(string=w2525, offset (0)=85, length (rest)=9 ("length (rest)")) -> (substring=w2528:string)
              n2046 = String Subset(string=w2525, offset (0)=35, length (rest)=9 ("length (rest)")) -> (substring=w2550:string)
              n2047 = String Subset(string=w2525, offset (0)=55, length (rest)=9 ("length (rest)")) -> (substring=w2536:string)
              n2048 = String Subset(string=w2525, offset (0)=25, length (rest)=9 ("length (rest)")) -> (substring=w2530:string)
              n2049 = String Subset(string=w2525, offset (0)=45, length (rest)=9 ("length (rest)")) -> (substring=w2538:string)
              n2050 = String Subset(string=w2525, offset (0)=0, length (rest)=14 ("length (rest)")) -> (substring=w2553:string)
              n2051 = String Subset(string=w2525, offset (0)=15, length (rest)=9 ("length (rest)")) -> (substring=w2556:string)
              n2052 = String Subset(string=w2525, offset (0)=65, length (rest)=9 ("length (rest)")) -> (substring=w2542:string)
              n2053 = Fract/Exp String To Number(string=w2528) -> (number=w2524:dbl)  [unwired: 3 in, 1 out]
              n2054 = Fract/Exp String To Number(string=w2550) -> (number=w2548:dbl)  [unwired: 3 in, 1 out]
              n2055 = Fract/Exp String To Number(string=w2536) -> (number=w2533:dbl)  [unwired: 3 in, 1 out]
              n2056 = Fract/Exp String To Number(string=w2530) -> (number=w2529:dbl)  [unwired: 3 in, 1 out]
              n2057 = Fract/Exp String To Number(string=w2538) -> (number=w2537:dbl)  [unwired: 3 in, 1 out]
              n2058 = Fract/Exp String To Number(string=w2553) -> (number=w2549:dbl)  [unwired: 3 in, 1 out]
              n2059 = Fract/Exp String To Number(string=w2556) -> (number=w2547:dbl)  [unwired: 3 in, 1 out]
              n2060 = Fract/Exp String To Number(string=w2542) -> (number=w2545:dbl)  [unwired: 3 in, 1 out]
              n2061 = Add(x=w2545, y=0.0) -> (x+y=w2541:dbl)
            }
            n2062 = for {
              N: w2433 -> [_]
              tunnel: w2440 -> [w2488]
              tunnel: w2439 -> [w2487]
              tunnel: [w2477] -> w2393 mode=indexing
              tunnel: [w2476] -> w2386 mode=indexing
              tunnel: w2430 -> [_]
              tunnel: [w2465] -> w2391 mode=indexing
              tunnel: [w2470] -> w2388 mode=indexing
              tunnel: [w2466] -> w2378 mode=indexing
              tunnel: [w2461] -> w2353 mode=indexing
              tunnel: [w2457] -> w2334 mode=indexing
              tunnel: [w2452] -> w2294 mode=indexing
              (unwired) 1.0 ("x")
              (unwired) TRUE ("line mode (F)")
              n2063 = Read from Text File "Read File"(file (use dialog)=w2488, error in=w2487) -> (text=w2453:string)  [unwired: 2 in, 3 out]
              n2064 = local write "String 12"(w2453) -> ()
              n2065 = String Subset(string=w2453, offset (0)=85, length (rest)=9 ("length (rest)")) -> (substring=w2455:string)
              n2066 = String Subset(string=w2453, offset (0)=35, length (rest)=9 ("length (rest)")) -> (substring=w2478:string)
              n2067 = String Subset(string=w2453, offset (0)=55, length (rest)=9 ("length (rest)")) -> (substring=w2463:string)
              n2068 = String Subset(string=w2453, offset (0)=25, length (rest)=9 ("length (rest)")) -> (substring=w2459:string)
              n2069 = String Subset(string=w2453, offset (0)=45, length (rest)=9 ("length (rest)")) -> (substring=w2468:string)
              n2070 = String Subset(string=w2453, offset (0)=15, length (rest)=9 ("length (rest)")) -> (substring=w2484:string)
              n2071 = String Subset(string=w2453, offset (0)=0, length (rest)=14 ("length (rest)")) -> (substring=w2481:string)
              n2072 = String Subset(string=w2453, offset (0)=65, length (rest)=9 ("length (rest)")) -> (substring=w2471:string)
              n2073 = Fract/Exp String To Number(string=w2455) -> (number=w2452:dbl)  [unwired: 3 in, 1 out]
              n2074 = Fract/Exp String To Number(string=w2478) -> (number=w2476:dbl)  [unwired: 3 in, 1 out]
              n2075 = Fract/Exp String To Number(string=w2463) -> (number=w2461:dbl)  [unwired: 3 in, 1 out]
              n2076 = Fract/Exp String To Number(string=w2459) -> (number=w2457:dbl)  [unwired: 3 in, 1 out]
              n2077 = Fract/Exp String To Number(string=w2468) -> (number=w2466:dbl)  [unwired: 3 in, 1 out]
              n2078 = Fract/Exp String To Number(string=w2484) -> (number=w2465:dbl)  [unwired: 3 in, 1 out]
              n2079 = Fract/Exp String To Number(string=w2481) -> (number=w2477:dbl)  [unwired: 3 in, 1 out]
              n2080 = Fract/Exp String To Number(string=w2471) -> (number=w2474:dbl)  [unwired: 3 in, 1 out]
              n2081 = Add(x=w2474, y=0.0) -> (x+y=w2470:dbl)
            }
            n2082 = Delete From Array(array=w2336, index=0) -> (array with subset deleted=w2309:dbl[])  [unwired: 1 in, 1 out]
            n2083 = Delete From Array(array=w2399, index=0) -> (array with subset deleted=w2372:dbl[])  [unwired: 1 in, 1 out]
            n2084 = Delete From Array(array=w2379, index=0) -> (array with subset deleted=w2367:dbl[])  [unwired: 1 in, 1 out]
            n2085 = Delete From Array(array=w2397, index=0) -> (array with subset deleted=w2398:dbl[])  [unwired: 1 in, 1 out]
            n2086 = call-poly <vilib>:"Mean.vi"("X"=w2309) -> ("mean"=→"КОФ2 4":dbl)  [unwired: 1 out]
            n2087 = call-poly <vilib>:"Mean.vi"("X"=w2372) -> ("mean"=→"КОФ3":dbl)  [unwired: 1 out]
            n2088 = call-poly <vilib>:"Mean.vi"("X"=w2367) -> ("mean"=→"CP3":dbl)  [unwired: 1 out]
            n2089 = Delete From Array(array=w2361, index=0) -> (array with subset deleted=w2288:dbl[])  [unwired: 1 in, 1 out]
            n2090 = Delete From Array(array=w2300, index=0) -> (array with subset deleted=w2287:dbl[])  [unwired: 1 in, 1 out]
            n2091 = Delete From Array(array=w2340, index=0) -> (array with subset deleted=w2311:dbl[])  [unwired: 1 in, 1 out]
            n2092 = Delete From Array(array=w2418, index=0) -> (array with subset deleted=w2373:dbl[])  [unwired: 1 in, 1 out]
            n2093 = Delete From Array(array=w2384, index=0) -> (array with subset deleted=w2369:dbl[])  [unwired: 1 in, 1 out]
            "array w/ subset deleted" <- w2369
            n2094 = Delete From Array(array=w2415, index=0) -> (array with subset deleted=w2416:dbl[])  [unwired: 1 in, 1 out]
            n2095 = call-poly <vilib>:"Mean.vi"("X"=w2311) -> ("mean"=→"КОФ2 2":dbl)  [unwired: 1 out]
            n2096 = call-poly <vilib>:"Mean.vi"("X"=w2373) -> ("mean"=→"КОФ1":dbl)  [unwired: 1 out]
            n2097 = Bundle "Bundle"(w2288, w2287) -> (w2293:cluster{dbl[], dbl[]})  [unwired: 1 in]
            n2098 = Bundle "Bundle"(w2288, w2416) -> (w2280:cluster{dbl[], dbl[]})  [unwired: 1 in]
            n2099 = Delete From Array(array=w2295, index=0) -> (array with subset deleted=w2283:dbl[])  [unwired: 1 in, 1 out]
            n2100 = Delete From Array(array=w2296, index=0) -> (array with subset deleted=w2285:dbl[])  [unwired: 1 in, 1 out]
            n2101 = Delete From Array(array=w2406, index=0) -> (array with subset deleted=w2407:dbl[])  [unwired: 1 in, 1 out]
            n2102 = Delete From Array(array=w2294, index=0) -> (array with subset deleted=w2281:dbl[])  [unwired: 1 in, 1 out]
            n2103 = Delete From Array(array=w2388, index=0) -> (array with subset deleted=w2389:dbl[])  [unwired: 1 in, 1 out]
            n2104 = Delete From Array(array=w2413, index=0) -> (array with subset deleted=w2319:dbl[])  [unwired: 1 in, 1 out]
            n2105 = Delete From Array(array=w2359, index=0) -> (array with subset deleted=w2315:dbl[])  [unwired: 1 in, 1 out]
            n2106 = Delete From Array(array=w2395, index=0) -> (array with subset deleted=w2317:dbl[])  [unwired: 1 in, 1 out]
            n2107 = Delete From Array(array=w2355, index=0) -> (array with subset deleted=w2313:dbl[])  [unwired: 1 in, 1 out]
            n2108 = Delete From Array(array=w2404, index=0) -> (array with subset deleted=w2318:dbl[])  [unwired: 1 in, 1 out]
            n2109 = Delete From Array(array=w2357, index=0) -> (array with subset deleted=w2314:dbl[])  [unwired: 1 in, 1 out]
            n2110 = Delete From Array(array=w2338, index=0) -> (array with subset deleted=w2310:dbl[])  [unwired: 1 in, 1 out]
            n2111 = Delete From Array(array=w2382, index=0) -> (array with subset deleted=w2368:dbl[])  [unwired: 1 in, 1 out]
            n2112 = Delete From Array(array=w2409, index=0) -> (array with subset deleted=w2370:dbl[])  [unwired: 1 in, 1 out]
            n2113 = Delete From Array(array=w2386, index=0) -> (array with subset deleted=w2316:dbl[])  [unwired: 1 in, 1 out]
            n2114 = Delete From Array(array=w2353, index=0) -> (array with subset deleted=w2312:dbl[])  [unwired: 1 in, 1 out]
            n2115 = Delete From Array(array=w2334, index=0) -> (array with subset deleted=w2308:dbl[])  [unwired: 1 in, 1 out]
            n2116 = Delete From Array(array=w2378, index=0) -> (array with subset deleted=w2366:dbl[])  [unwired: 1 in, 1 out]
            n2117 = Delete From Array(array=w2391, index=0) -> (array with subset deleted=w2371:dbl[])  [unwired: 1 in, 1 out]
            n2118 = Delete From Array(array=w2401, index=0) -> (array with subset deleted=w2284:dbl[])  [unwired: 1 in, 1 out]
            n2119 = Delete From Array(array=w2411, index=0) -> (array with subset deleted=w2286:dbl[])  [unwired: 1 in, 1 out]
            n2120 = Delete From Array(array=w2393, index=0) -> (array with subset deleted=w2282:dbl[])  [unwired: 1 in, 1 out]
            n2121 = Bundle "Bundle"(w2288, w2319) -> (w2306:cluster{dbl[], dbl[]})  [unwired: 1 in]
            n2122 = Bundle "Bundle"(w2288, w2373) -> (w2307:cluster{dbl[], dbl[]})  [unwired: 1 in]
            n2123 = Bundle "Bundle"(w2319, w2315) -> (w2321:cluster{dbl[], dbl[]})  [unwired: 1 in]
            n2124 = Bundle "Bundle"(w2284, w2283) -> (w2291:cluster{dbl[], dbl[]})  [unwired: 1 in]
            n2125 = Bundle "Bundle"(w2317, w2313) -> (w2323:cluster{dbl[], dbl[]})  [unwired: 1 in]
            n2126 = Bundle "Bundle"(w2284, w2317) -> (w2427:cluster{dbl[], dbl[]})  [unwired: 1 in]
            n2127 = Bundle "Bundle"(w2284, w2313) -> (w2351:cluster{dbl[], dbl[]})  [unwired: 1 in]
            n2128 = Bundle "Bundle"(w2284, w2372) -> (w2437:cluster{dbl[], dbl[]})  [unwired: 1 in]
            n2129 = Bundle "Bundle"(w2284, w2367) -> (w2375:cluster{dbl[], dbl[]})  [unwired: 1 in]
            n2130 = Bundle "Bundle"(w2284, w2398) -> (w2422:cluster{dbl[], dbl[]})  [unwired: 1 in]
            n2131 = Bundle "Bundle"(w2318, w2314) -> (w2322:cluster{dbl[], dbl[]})  [unwired: 1 in]
            n2132 = Bundle "Bundle"(w2286, w2285) -> (w2292:cluster{dbl[], dbl[]})  [unwired: 1 in]
            n2133 = Bundle "Bundle"(w2286, w2318) -> (w2429:cluster{dbl[], dbl[]})  [unwired: 1 in]
            n2134 = Bundle "Bundle"(w2286, w2314) -> (w2352:cluster{dbl[], dbl[]})  [unwired: 1 in]
            n2135 = Bundle "Bundle"(w2286, w2368) -> (w2376:cluster{dbl[], dbl[]})  [unwired: 1 in]
            n2136 = Bundle "Bundle"(w2286, w2370) -> (w2438:cluster{dbl[], dbl[]})  [unwired: 1 in]
            n2137 = Bundle "Bundle"(w2286, w2407) -> (w2420:cluster{dbl[], dbl[]})  [unwired: 1 in]
            n2138 = Bundle "Bundle"(w2316, w2312) -> (w2324:cluster{dbl[], dbl[]})  [unwired: 1 in]
            n2139 = Bundle "Bundle"(w2282, w2281) -> (w2290:cluster{dbl[], dbl[]})  [unwired: 1 in]
            n2140 = Bundle "Bundle"(w2282, w2316) -> (w2428:cluster{dbl[], dbl[]})  [unwired: 1 in]
            n2141 = Bundle "Bundle"(w2282, w2312) -> (w2350:cluster{dbl[], dbl[]})  [unwired: 1 in]
            n2142 = Bundle "Bundle"(w2282, w2366) -> (w2374:cluster{dbl[], dbl[]})  [unwired: 1 in]
            n2143 = Bundle "Bundle"(w2282, w2371) -> (w2436:cluster{dbl[], dbl[]})  [unwired: 1 in]
            n2144 = Bundle "Bundle"(w2282, w2389) -> (w2421:cluster{dbl[], dbl[]})  [unwired: 1 in]
            n2145 = call-poly <vilib>:"Mean.vi"("X"=w2369) -> ("mean"=→"CP1":dbl)  [unwired: 1 out]
            n2146 = call-poly <vilib>:"Mean.vi"("X"=w2310) -> ("mean"=→"КОФ2 3":dbl)  [unwired: 1 out]
            n2147 = call-poly <vilib>:"Mean.vi"("X"=w2368) -> ("mean"=→"CP2":dbl)  [unwired: 1 out]
            n2148 = call-poly <vilib>:"Mean.vi"("X"=w2370) -> ("mean"=→"КОФ2":dbl)  [unwired: 1 out]
            n2149 = call-poly <vilib>:"Mean.vi"("X"=w2308) -> ("mean"=→"КОФ2 5":dbl)  [unwired: 1 out]
            n2150 = call-poly <vilib>:"Mean.vi"("X"=w2366) -> ("mean"=→"CP4":dbl)  [unwired: 1 out]
            n2151 = call-poly <vilib>:"Mean.vi"("X"=w2371) -> ("mean"=→"КОФ4":dbl)  [unwired: 1 out]
            n2152 = Bundle "Bundle"(w2288, w2315) -> (w2279:cluster{dbl[], dbl[]})  [unwired: 1 in]
            n2153 = Bundle "Bundle"(w2288, w2369) -> (w2302:cluster{dbl[], dbl[]})  [unwired: 1 in]
            n2154 = Build Array "Build Array"(w2279, w2302) -> (w2305:cluster{dbl[], dbl[]}[])
            "XY Graph 17" <- w2305
            n2155 = Build Array "Build Array"(w2293, w2292, w2291, w2290) -> (→"Frequency ( Hz )":cluster{dbl[], dbl[]}[])
            n2156 = Build Array "Build Array"(w2321, w2322, w2323, w2324) -> (→"Air Temp ( °C ) vs Humidity ( % RH )":cluster{dbl[], dbl[]}[])
            n2157 = Build Array "Build Array"(w2306, w2429, w2427, w2428) -> (→"Air Temperature  ( °C )":cluster{dbl[], dbl[]}[])
            n2158 = Build Array "Build Array"(w2279, w2352, w2351, w2350) -> (→"Humidity ( %RH )":cluster{dbl[], dbl[]}[])
            n2159 = Build Array "Build Array"(w2307, w2438, w2437, w2436) -> (→"Coefficient Of Friction":cluster{dbl[], dbl[]}[])
            n2160 = Build Array "Build Array"(w2302, w2376, w2375, w2374) -> (→"Sample Temperature ( °C )":cluster{dbl[], dbl[]}[])
            n2161 = Build Array "Build Array"(w2280, w2420, w2422, w2421) -> (→"XY Graph 13":cluster{dbl[], dbl[]}[])
            n2162 = Bundle "Bundle"(w2288, w2311) -> (w2333:cluster{dbl[], dbl[]})  [unwired: 1 in]
            n2163 = Bundle "Bundle"(w2284, w2309) -> (w2331:cluster{dbl[], dbl[]})  [unwired: 1 in]
            n2164 = Bundle "Bundle"(w2286, w2310) -> (w2332:cluster{dbl[], dbl[]})  [unwired: 1 in]
            n2165 = Bundle "Bundle"(w2282, w2308) -> (w2330:cluster{dbl[], dbl[]})  [unwired: 1 in]
            n2166 = Build Array "Build Array"(w2333, w2332, w2331, w2330) -> (→"Stroke ( mm )":cluster{dbl[], dbl[]}[])
            n2167 = local write "XY Graph 16"(w2305) -> ()
          }
          frame #2 {
          }
          frame #3 {
            n2168 = local write "Numeric 8"(0 ("Numeric 8")) -> ()
            n2169 = local write "Numeric 11"(0 ("Numeric 11")) -> ()
            n2170 = local write "Numeric 12"(0 ("Numeric 12")) -> ()
            n2171 = local write "Numeric 13"(0 ("Numeric 13")) -> ()
            n2172 = property on="OPEN" class="Bool (strict)"("Visible"=TRUE) -> ()  [unwired: 2 in, 2 out]
            n2173 = local read "String Control 2"() -> (w2605:string)
            n2174 = local read "String Control 4"() -> (w2604:string)
            n2175 = local read "String Control 6"() -> (w2603:string)
            n2176 = local read "String Control 8"() -> (w2602:string)
            n2177 = Match Pattern(string=w2605, regular expression="Samples / cycle :- ") -> (after substring=w2619:string)  [unwired: 1 in, 3 out]
            n2178 = Match Pattern(string=w2605, regular expression="Frequency :- ") -> (after substring=w2638:string)  [unwired: 1 in, 3 out]
            n2179 = Match Pattern(string=w2604, regular expression="Samples / cycle :- ") -> (after substring=w2615:string)  [unwired: 1 in, 3 out]
            n2180 = Match Pattern(string=w2604, regular expression="Frequency :- ") -> (after substring=w2633:string)  [unwired: 1 in, 3 out]
            n2181 = Match Pattern(string=w2603, regular expression="Samples / cycle :- ") -> (after substring=w2611:string)  [unwired: 1 in, 3 out]
            n2182 = Match Pattern(string=w2603, regular expression="Frequency :- ") -> (after substring=w2628:string)  [unwired: 1 in, 3 out]
            n2183 = Match Pattern(string=w2602, regular expression="Samples / cycle :- ") -> (after substring=w2607:string)  [unwired: 1 in, 3 out]
            n2184 = Match Pattern(string=w2602, regular expression="Frequency :- ") -> (after substring=w2623:string)  [unwired: 1 in, 3 out]
            n2185 = String Subset(string=w2619, length (rest)=6 ("length (rest)")) -> (substring=w2621:string)  [unwired: 1 in]